vi "Main.vi"() -> ()   [LabVIEW 2018] (continued)
                n1059 = call "DrawROICircle.vi"("old picture"=w1988, "ROI?"=w1976, "Radius (G/S)"=w1975, "Center (G/S)"=w1974, "PicSize"=w1990, "Color"=w1973, "G_max"=w1970, "S_max"=w1968, "G_min"=w1969, "S_min"=w1967) -> ("new picture"=w1987:picture)  [unwired: 9 in]
                n1060 = case shown="\"ROI4\"" w1992 {
                  tunnel: w1993 -> [_ w2002 w2003 w2004 w2005]
                  frame "None" {
                  }
                  frame "ROI1" {
                    "Radius1" <- w2002
                  }
                  frame "ROI2" {
                    "Radius2" <- w2003
                  }
                  frame "ROI3" {
                    "Radius3" <- w2004
                  }
                  frame "ROI4" {
                    "Radius4" <- w2005
                  }
                }
              }
            }
          }
        }
        n1061 = property on="Phasor Plot" class="IntGraph (strict)"(error in=w1891, "PlotImages.Front"=w1892) -> (error out=w1897:errorcluster)  [unwired: 1 in, 1 out]
      }
      event "Phasor Plot": Mouse Up; "ROI1?", "ROI2?", "ROI3?", "ROI4?", "Phasor\nOverlap?", "Refresh Overlap": Value Change {
        n1062 = event-data() -> ()  [unwired: 1 in, 1 out]
        n1063 = local read "ROI Drawing"() -> (w2050:bool)
        n1064 = local read "ROI Select"() -> (w2051:enum16{"None", "ROI1", "ROI2", "ROI3", "ROI4"})
        n1065 = case shown="True" w2050 {
          tunnel: w2051 -> [_ w2076]
          tunnel: w2043 -> [w2073 w2074]
          tunnel: [w2073 w2074] -> w2042
          frame False {
          }
          frame True {
            n1066 = case shown="\"ROI1\"" w2076 {
              frame "None" {
              }
              frame "ROI1" {
                n1067 = local read "Radius1"() -> (w2081:dbl)
                n1068 = Greater Than 0?(x=w2081) -> (x > 0?=w2080:bool)
                n1069 = Select(t=TRUE ("ROI Drawing"), s=w2080, f=FALSE ("ROI Drawing")) -> (s? t:f=w2079:bool)
                n1070 = local write "ROI1?"(w2079) -> ()
              }
              frame "ROI2" {
                n1071 = local read "Radius2"() -> (w2083:dbl)
                n1072 = Greater Than 0?(x=w2083) -> (x > 0?=w2086:bool)
                n1073 = Select(t=TRUE ("ROI Drawing"), s=w2086, f=FALSE ("ROI Drawing")) -> (s? t:f=w2082:bool)
                n1074 = local write "ROI2?"(w2082) -> ()
              }
              frame "ROI3" {
                n1075 = local read "Radius3"() -> (w2089:dbl)
                n1076 = Greater Than 0?(x=w2089) -> (x > 0?=w2090:bool)
                n1077 = Select(t=TRUE ("ROI Drawing"), s=w2090, f=FALSE ("ROI Drawing")) -> (s? t:f=w2088:bool)
                n1078 = local write "ROI3?"(w2088) -> ()
              }
              frame "ROI4" {
                n1079 = local read "Radius4"() -> (w2093:dbl)
                n1080 = Greater Than 0?(x=w2093) -> (x > 0?=w2096:bool)
                n1081 = Select(t=TRUE ("ROI Drawing"), s=w2096, f=FALSE ("ROI Drawing")) -> (s? t:f=w2092:bool)
                n1082 = local write "ROI4?"(w2092) -> ()
              }
            }
            n1083 = local write "ROI Drawing"(FALSE ("ROI Drawing")) -> ()
          }
        }
        n1084 = local read "Radius4"() -> (w2038:dbl)
        n1085 = local read "Center4"() -> (w2035:cluster{dbl, dbl})
        n1086 = local read "Radius2"() -> (w2040:dbl)
        n1087 = local read "Center2"() -> (w2036:cluster{dbl, dbl})
        n1088 = local read "Radius3"() -> (w2039:dbl)
        n1089 = local read "Center3"() -> (w2026:cluster{dbl, dbl})
        n1090 = local read "Radius1"() -> (w2041:dbl)
        n1091 = local read "Center1"() -> (w2037:cluster{dbl, dbl})
        n1092 = local read "PicSize"() -> (w2046:u32)
        n1093 = local read "Color4"() -> (w2031:u32)
        n1094 = local read "Color2"() -> (w2033:u32)
        n1095 = local read "Color3"() -> (w2032:u32)
        n1096 = local read "Color1"() -> (w2034:u32)
        n1097 = local read "ROI4?"() -> (w2016:bool)
        n1098 = local read "ROI3?"() -> (w2017:bool)
        n1099 = local read "ROI1?"() -> (w2019:bool)
        n1100 = local read "ROI2?"() -> (w2018:bool)
        n1101 = Build Array(w2019, w2018, w2017, w2016) -> (w2015:bool[])
        n1102 = Build Array(w2041, w2040, w2039, w2038) -> (w2014:dbl[])
        n1103 = Build Array(w2037, w2036, w2026, w2035) -> (w2013:cluster{dbl, dbl}[])
        n1104 = local read "G_max"() -> (w2025:dbl)
        n1105 = local read "G_min"() -> (w2024:dbl)
        n1106 = local read "S_max"() -> (w2023:dbl)
        n1107 = Build Array(w2034, w2033, w2032, w2031) -> (w2012:u32[])
        n1108 = local read "S_min"() -> (w2022:dbl)
        n1109 = call "Empty Picture"() -> ("empty picture"=w2044:picture)
        n1110 = call "DrawROICircle.vi"("old picture"=w2044, "ROI?"=w2019, "Radius (G/S)"=w2041, "Center (G/S)"=w2037, "PicSize"=w2046, "Color"=w2034, "G_max"=w2025, "S_max"=w2023, "G_min"=w2024, "S_min"=w2022) -> ("new picture"=w2049:picture)  [unwired: 9 in]
        n1111 = call "DrawROICircle.vi"("old picture"=w2049, "ROI?"=w2018, "Radius (G/S)"=w2040, "Center (G/S)"=w2036, "PicSize"=w2046, "Color"=w2033, "G_max"=w2025, "S_max"=w2023, "G_min"=w2024, "S_min"=w2022) -> ("new picture"=w2047:picture)  [unwired: 9 in]
        n1112 = call "DrawROICircle.vi"("old picture"=w2047, "ROI?"=w2017, "Radius (G/S)"=w2039, "Center (G/S)"=w2026, "PicSize"=w2046, "Color"=w2032, "G_max"=w2025, "S_max"=w2023, "G_min"=w2024, "S_min"=w2022) -> ("new picture"=w2048:picture)  [unwired: 9 in]
        n1113 = call "DrawROICircle.vi"("old picture"=w2048, "ROI?"=w2016, "Radius (G/S)"=w2038, "Center (G/S)"=w2035, "PicSize"=w2046, "Color"=w2031, "G_max"=w2025, "S_max"=w2023, "G_min"=w2024, "S_min"=w2022) -> ("new picture"=w2045:picture)  [unwired: 9 in]
        n1114 = local read "Auto Scale?"() -> (w2010:bool)
        n1115 = local read "Max Intensity"() -> (w2009:dbl)
        n1116 = local read "Min Intensity"() -> (w2008:dbl)
        n1117 = control-ref of="Image with Phasors"() -> (w2028:refnum<vi>)
        n1118 = property on="Phasor Plot" class="IntGraph (strict)"(error in=w2042, "PlotImages.Front"=w2045) -> (error out=w2021:errorcluster)  [unwired: 1 in, 1 out]
        n1119 = Bundle(w2015, w2014, w2013, w2012) -> (→"ROI Cluster":T9)  [unwired: 1 in]
        n1120 = local read "V_DC"() -> (w2027:dbl[][])
        n1121 = case shown="True" "Phasor\nOverlap?" {
          tunnel: w2015 -> [_ w2070]
          tunnel: w2014 -> [_ w2069]
          tunnel: w2013 -> [_ w2068]
          tunnel: w2012 -> [_ w2067]
          tunnel: [w2060 w2066] -> w2029
          tunnel: w2028 -> [w2059 w2065]
          tunnel: w2010 -> [w2057 w2064]
          tunnel: w2009 -> [w2056 w2063]
          tunnel: w2008 -> [w2055 w2062]
          tunnel: w2027 -> [w2058 w2061]
          frame False {
            n1122 = call "Array2GrayPic.vi"("Pic Reference"=w2059, "Threshold (min)"=w2055, "Threshold (max)"=w2056, "Auto Scale?"=w2057, "Intensity"=w2058) -> ("Gray Picture"=w2060:picture)  [unwired: 6 in]
          }
          frame True {
            n1123 = local read "G Data"() -> (w2072:dbl[][])
            n1124 = local read "S Data"() -> (w2071:dbl[][])
            n1125 = call "PhasorROI2IMG.vi"("Intensity"=w2061, "Auto Scale?"=w2064, "Threshold (max)"=w2063, "Threshold (min)"=w2062, "G Data"=w2072, "S Data"=w2071, "Pic Reference"=w2065, "ROI? array"=w2070, "Radius array"=w2069, "Center array"=w2068, "Color array"=w2067) -> ("new picture"=w2066:picture)  [unwired: 8 in]
          }
        }
        n1126 = flat-sequence {
          tunnel: [w2054] -> w2020
          tunnel: w2021 -> [w2054]
          frame #0 {
            n1127 = local write "Refresh Overlap"(FALSE ("Fast Scan")) -> ()
          }
        }
        n1128 = local write "Image with Phasors"(w2029) -> ()
      }
      event "Phasor Grids", "G_max", "G_min", "S_max", "S_min", "Phasor Colormap", "Update Phasor": Value Change {
        n1129 = event-data() -> ()  [unwired: 1 in, 1 out]
        n1130 = local read "Phasor Colormap"() -> (w2102:T8)
        n1131 = local read "Max Intensity"() -> (w2100:dbl)
        n1132 = local read "Min Intensity"() -> (w2099:dbl)
        n1133 = local read "Auto Scale?"() -> (w2101:bool)
        n1134 = control-ref of="Phasor Plot"() -> (w2103:refnum<vi>)
        n1135 = local read "Phasor Grids"() -> (w2104:i32)
        n1136 = local read "V_DC"() -> (w2107:dbl[][])
        n1137 = control-ref of="Image with Phasors"() -> (w2116:refnum<vi>)
        n1138 = local read "G Data"() -> (w2106:dbl[][])
        n1139 = local read "S Data"() -> (w2105:dbl[][])
        n1140 = local read "G_max"() -> (w2111:dbl)
        n1141 = local read "S_max"() -> (w2109:dbl)
        n1142 = local read "G_min"() -> (w2110:dbl)
        n1143 = local read "S_min"() -> (w2108:dbl)
        n1144 = call "Array2GrayPic.vi"("Pic Reference"=w2116, "Threshold (min)"=w2099, "Threshold (max)"=w2100, "Auto Scale?"=w2101, "Intensity"=w2107) -> ("Gray Picture"=w2115:picture)  [unwired: 6 in]
        n1145 = call "DrawPhasorPlot.vi"("Intensity"=w2107, "G Data"=w2106, "S Data"=w2105, "Threshold (max)"=w2100, "Threshold (min)"=w2099, "error in"=w2114, "G_max"=w2111, "Auto Scale?"=w2101, "G_min"=w2110, "Phasor Grids"=w2104, "S_max"=w2109, "Reference"=w2103, "S_min"=w2108, "Phasor Colormap"=w2102) -> ("Phasor Plot"=w2112:dbl[][], "error out"=w2113:errorcluster)  [unwired: 4 in]
        n1146 = local write "Image with Phasors"(w2115) -> ()
        n1147 = local write "Phasor Plot"(w2112) -> ()
      }
      event "Load P1": Value Change {
        n1148 = event-data() -> ()  [unwired: 1 in, 1 out]
        n1149 = local read "Measurement Parameters"() -> (w2138:T4)
        n1150 = property on="Composite q1,1" class="Pict"(error in=w2135) -> (error out=w2134:errorcluster, "Draw Area Size"=w2139:T16)  [unwired: 1 in, 1 out]
        n1151 = local read "V_DC"() -> (→"DC,1":dbl[][])
        n1152 = local read "V_IF (pi)"() -> (w2159:dbl[][])
        n1153 = local read "V_IF (0)"() -> (w2158:dbl[][])
        n1154 = local read "V_IF (0.5pi)"() -> (w2157:dbl[][])
        n1155 = local read "V_IF (1.5pi)"() -> (w2156:dbl[][])
        n1156 = Unbundle By Name(w2138) -> ("Pixel Size"=w2137:dbl)
        n1157 = Unbundle By Name(w2139) -> ("Width"=w2140:u32)
        n1158 = To Single Precision Float(number=w2140) -> (single precision float=w2142:sgl)
        n1159 = To Single Precision Float(number=w2137) -> (single precision float=w2141:sgl)
        n1160 = Divide(x=w2142, y=w2141) -> (x/y=w2136:sgl)
        n1161 = Subtract(x=w2159, y=w2158) -> (x-y=w2151:dbl[][])
        n1162 = Subtract(x=w2157, y=w2156) -> (x-y=w2152:dbl[][])
        n1163 = property on="Composite q1,1" class="Pict"(error in=w2134, "ZoomFactor"=w2136) -> (error out=w2130:errorcluster)  [unwired: 1 in, 1 out]
        n1164 = local read "tau_max (s)"() -> (w2132:dbl)
        n1165 = local read "tau_min (s)"() -> (w2131:dbl)
        n1166 = Square(x=w2151) -> (x^2=w2155:dbl[][])
        n1167 = Square(x=w2152) -> (x^2=w2154:dbl[][])
        n1168 = Divide(x=w2151, y=w2152) -> (x/y=w2150:dbl[][])
        n1169 = local read "LaserRepRate (Hz)"() -> (w2118:dbl)
        n1170 = Add(x=w2155, y=w2154) -> (x+y=w2153:dbl[][])
        n1171 = Inverse Tangent(1:w2150) -> (0:w2148:dbl[][])
        "Angle q1,1" <- w2148
        n1172 = property on="Lifetime q1,1" class="IntGraph (strict)"(error in=w2130, "ZScale.Minimum"=w2131) -> (error out=w2129:errorcluster)  [unwired: 1 in, 1 out]
        n1173 = Square Root(x=w2153) -> (sqrt(x)=w2127:dbl[][])
        "Mag q1,1" <- w2127
        n1174 = Tangent(1:w2148) -> (0:w2147:dbl[][])
        n1175 = Multiply(x=w2118, y=6.283185307179586) -> (x*y=w2146:dbl)
        n1176 = local read "Custom Mag?"() -> (w2128:bool)
        n1177 = Divide(x=w2147, y=w2146) -> (x/y=w2145:dbl[][])
        n1178 = property on="Lifetime q1,1" class="IntGraph (strict)"(error in=w2129, "ZScale.Maximum"=w2132) -> (error out=w2126:errorcluster)  [unwired: 1 in, 1 out]
        n1179 = Negate(x=w2145) -> (-x=w2143:dbl[][])
        "Lifetime q1,1" <- w2143
        n1180 = case shown="True" w2128 {
          tunnel: w2127 -> [w2163 _]
          tunnel: [w2162 "q1,1max"] -> w2122
          tunnel: [w2161 "q1,1min"] -> w2123
          frame False {
            n1181 = Array Max & Min(array=w2163) -> (max value=w2162:dbl, min value=w2161:dbl)  [unwired: 2 out]
          }
          frame True {
          }
        }
        n1182 = call "HSVCombIntensityLifetime.vi"("min_intensity"=w2123, "Auto Scale?"=TRUE ("External Bound Intensity Value?"), "max_intensity"=w2122, "lifetime_max (s)"=w2132, "lifetime_min (s)"=w2131, "Lifetime image"=w2143, "Intensity image"=w2127) -> ("HSV to RGB Picture"=→"Composite q1,1":picture)  [unwired: 1 in, 3 out]
        n1183 = property on="Mag q1,1" class="IntGraph (strict)"(error in=w2126, "ZScale.Minimum"=w2123) -> (error out=w2125:errorcluster)  [unwired: 1 in, 1 out]
        n1184 = property on="Mag q1,1" class="IntGraph (strict)"(error in=w2125, "ZScale.Maximum"=w2122) -> (error out=w2124:errorcluster)  [unwired: 1 in, 1 out]
      }
      event "Load P2": Value Change {
        n1185 = event-data() -> ()  [unwired: 1 in, 1 out]
        n1186 = local read "Measurement Parameters"() -> (w2186:T4)
        n1187 = property on="Composite q1,2" class="Pict"(error in=w2185) -> (error out=w2184:errorcluster, "Draw Area Size"=w2183:T16)  [unwired: 1 in, 1 out]
        n1188 = Unbundle By Name(w2186) -> ("Pixel Size"=w2187:dbl)
        n1189 = local read "V_IF (pi)"() -> (w2201:dbl[][])
        n1190 = local read "V_IF (0)"() -> (w2200:dbl[][])
        n1191 = local read "V_IF (0.5pi)"() -> (w2199:dbl[][])
        n1192 = local read "V_IF (1.5pi)"() -> (w2198:dbl[][])
        n1193 = local read "V_DC"() -> (→"DC,2":dbl[][])
        n1194 = Unbundle By Name(w2183) -> ("Width"=w2188:u32)
        n1195 = To Single Precision Float(number=w2188) -> (single precision float=w2190:sgl)
        n1196 = To Single Precision Float(number=w2187) -> (single precision float=w2189:sgl)
        n1197 = Divide(x=w2190, y=w2189) -> (x/y=w2182:sgl)
        n1198 = Subtract(x=w2201, y=w2200) -> (x-y=w2203:dbl[][])
        n1199 = Subtract(x=w2199, y=w2198) -> (x-y=w2204:dbl[][])
        n1200 = property on="Composite q1,2" class="Pict"(error in=w2184, "ZoomFactor"=w2182) -> (error out=w2177:errorcluster)  [unwired: 1 in, 1 out]
        n1201 = local read "tau_max (s)"() -> (w2180:dbl)
        n1202 = local read "tau_min (s)"() -> (w2181:dbl)
        n1203 = Square(x=w2203) -> (x^2=w2207:dbl[][])
        n1204 = Square(x=w2204) -> (x^2=w2206:dbl[][])
        n1205 = Divide(x=w2203, y=w2204) -> (x/y=w2202:dbl[][])
        n1206 = property on="Lifetime q1,2" class="IntGraph (strict)"(error in=w2177, "ZScale.Minimum"=w2181) -> (error out=w2176:errorcluster)  [unwired: 1 in, 1 out]
        n1207 = local read "LaserRepRate (Hz)"() -> (w2166:dbl)
        n1208 = Add(x=w2207, y=w2206) -> (x+y=w2205:dbl[][])
        n1209 = Inverse Tangent(1:w2202) -> (0:w2170:dbl[][])
        "Angle q1,2" <- w2170
        n1210 = local read "Custom Mag?"() -> (w2179:bool)
        n1211 = property on="Lifetime q1,2" class="IntGraph (strict)"(error in=w2176, "ZScale.Maximum"=w2180) -> (error out=w2175:errorcluster)  [unwired: 1 in, 1 out]
        n1212 = Square Root(x=w2205) -> (sqrt(x)=w2178:dbl[][])
        "Mag q1,2" <- w2178
        n1213 = Tangent(1:w2170) -> (0:w2196:dbl[][])
        n1214 = Multiply(x=w2166, y=6.283185307179586) -> (x*y=w2195:dbl)
        n1215 = case shown="True" w2179 {
          tunnel: w2178 -> [w2211 _]
          tunnel: [w2210 "q1,2max"] -> w2172
          tunnel: [w2209 "q1,2min"] -> w2171
          frame False {
            n1216 = Array Max & Min(array=w2211) -> (max value=w2210:dbl, min value=w2209:dbl)  [unwired: 2 out]
          }
          frame True {
          }
        }
        n1217 = Divide(x=w2196, y=w2195) -> (x/y=w2194:dbl[][])
        n1218 = Negate(x=w2194) -> (-x=w2192:dbl[][])
        "Lifetime q1,2" <- w2192
        n1219 = call "HSVCombIntensityLifetime.vi"("min_intensity"=w2171, "Auto Scale?"=TRUE ("External Bound Intensity Value?"), "max_intensity"=w2172, "lifetime_max (s)"=w2180, "lifetime_min (s)"=w2181, "Lifetime image"=w2192, "Intensity image"=w2178) -> ("HSV to RGB Picture"=→"Composite q1,2":picture)  [unwired: 1 in, 3 out]
        n1220 = property on="Mag q1,2" class="IntGraph (strict)"(error in=w2175, "ZScale.Minimum"=w2171) -> (error out=w2174:errorcluster)  [unwired: 1 in, 1 out]
        n1221 = property on="Mag q1,2" class="IntGraph (strict)"(error in=w2174, "ZScale.Maximum"=w2172) -> (error out=w2173:errorcluster)  [unwired: 1 in, 1 out]
      }
      event "Two-Step GSOS": Value Change {
        n1222 = event-data() -> ()  [unwired: 1 in, 1 out]
        n1223 = local read "Measurement Parameters"() -> (w2237:T4)
        n1224 = property on="Composite GSOS" class="Pict"(error in=w2239) -> (error out=w2238:errorcluster, "Draw Area Size"=w2241:T16)  [unwired: 1 in, 1 out]
        n1225 = local read "Mag q1,1"() -> (w2262:dbl[][])
        n1226 = local read "Angle q1,2"() -> (w2224:dbl[][])
        n1227 = local read "Angle q1,1"() -> (w2225:dbl[][])
        n1228 = local read "Mag q1,2"() -> (w2261:dbl[][])
        n1229 = local read "DC,1"() -> (w2220:dbl[][])
        n1230 = local read "DC,2"() -> (w2222:dbl[][])
        n1231 = Unbundle By Name(w2237) -> ("Pixel Size"=w2242:dbl)
        n1232 = Unbundle By Name(w2241) -> ("Width"=w2243:u32)
        n1233 = To Single Precision Float(number=w2243) -> (single precision float=w2245:sgl)
        n1234 = To Single Precision Float(number=w2242) -> (single precision float=w2244:sgl)
        n1235 = Divide(x="P1 Power (au)", y="P2 Power (au)") -> (x/y=w2258:dbl)
        n1236 = Polar To Complex(1:w2224, 2:w2261) -> (0:w2255:cdb[][])
        n1237 = Polar To Complex(1:w2225, 2:w2262) -> (0:w2256:cdb[][])
        n1238 = Square(x=w2258) -> (x^2=w2257:dbl)
        n1239 = Divide(x=w2245, y=w2244) -> (x/y=w2240:sgl)
        n1240 = Negate(x=w2257) -> (-x=w2219:dbl)
        n1241 = property on="Composite GSOS" class="Pict"(error in=w2238, "ZoomFactor"=w2240) -> (error out=w2234:errorcluster)  [unwired: 1 in, 1 out]
        n1242 = To Double Precision Complex(1:w2219) -> (0:w2221:cdb)
        n1243 = local read "tau_max (s)"() -> (w2235:dbl)
        n1244 = local read "tau_min (s)"() -> (w2236:dbl)
        n1245 = Multiply(x=w2255, y=w2221) -> (x*y=w2254:cdb[][])
        n1246 = Multiply(x=w2222, y=w2219) -> (x*y=w2218:dbl[][])
        n1247 = Add(x=w2220, y=w2218) -> (x+y=→"DC,SOS":dbl[][])
        n1248 = Add(x=w2256, y=w2254) -> (x+y=w2253:cdb[][])
        n1249 = property on="Lifetime GSOS" class="IntGraph (strict)"(error in=w2234, "ZScale.Minimum"=w2236) -> (error out=w2233:errorcluster)  [unwired: 1 in, 1 out]
        n1250 = local read "LaserRepRate (Hz)"() -> (w2214:dbl)
        n1251 = Complex To Polar(r * e^(i*theta)=w2253) -> (r=w2231:dbl[][], theta=w2223:dbl[][])
        "Mag GSOS" <- w2231
        "Angle GSOS" <- w2223
        n1252 = local read "Custom Mag?"() -> (w2232:bool)
        n1253 = property on="Lifetime GSOS" class="IntGraph (strict)"(error in=w2233, "ZScale.Maximum"=w2235) -> (error out=w2230:errorcluster)  [unwired: 1 in, 1 out]
        n1254 = Tangent(1:w2223) -> (0:w2251:dbl[][])
        n1255 = case shown="True" w2232 {
          tunnel: w2231 -> [w2266 _]
          tunnel: [w2265 "qGSmax"] -> w2227
          tunnel: [w2264 "qGSmin"] -> w2226
          frame False {
            n1256 = Array Max & Min(array=w2266) -> (max value=w2265:dbl, min value=w2264:dbl)  [unwired: 2 out]
          }
          frame True {
          }
        }
        n1257 = Multiply(x=w2214, y=6.283185307179586) -> (x*y=w2250:dbl)
        n1258 = Divide(x=w2251, y=w2250) -> (x/y=w2249:dbl[][])
        n1259 = Negate(x=w2249) -> (-x=w2247:dbl[][])
        "Lifetime GSOS" <- w2247
        n1260 = call "HSVCombIntensityLifetime.vi"("min_intensity"=w2226, "Auto Scale?"=TRUE ("External Bound Intensity Value?"), "max_intensity"=w2227, "lifetime_max (s)"=w2235, "lifetime_min (s)"=w2236, "Lifetime image"=w2247, "Intensity image"=w2231) -> ("HSV to RGB Picture"=→"Composite GSOS":picture)  [unwired: 1 in, 3 out]
        n1261 = property on="Mag GSOS" class="IntGraph (strict)"(error in=w2230, "ZScale.Minimum"=w2226) -> (error out=w2229:errorcluster)  [unwired: 1 in, 1 out]
        n1262 = property on="Mag GSOS" class="IntGraph (strict)"(error in=w2229, "ZScale.Maximum"=w2227) -> (error out=w2228:errorcluster)  [unwired: 1 in, 1 out]
      }
      event "Export GSOS Images": Value Change {
        n1263 = event-data() -> ()  [unwired: 1 in, 1 out]
        n1264 = local read "Current Directory (2D)?"() -> (w2349:bool)
        n1265 = local read "Mag q1,1"() -> (w2315:dbl[][])
        n1266 = local read "Mag q1,2"() -> (w2314:dbl[][])
        n1267 = local read "Mag GSOS"() -> (w2313:dbl[][])
        n1268 = case shown="True" w2349 {
          tunnel: [w2373 w2374] -> w2348
          frame False {
            n1269 = local read "Save Directory (2D)"() -> (w2373:path)
          }
          frame True {
            n1270 = Current VI's Path() -> (path=w2375:path)
            n1271 = Strip Path(path=w2375) -> (stripped path=w2374:path)  [unwired: 1 out]
          }
        }
        n1272 = local read "Experiment Name (2D)"() -> (w2347:string)
        n1273 = local read "File Name (2D)"() -> (w2322:string)
        n1274 = case shown="True" "Custom Mag?" {
          tunnel: w2315 -> [w2366 _]
          tunnel: [w2365 w2372] -> w2312
          tunnel: [w2364 w2371] -> w2311
          tunnel: [w2362 w2370] -> w2310
          tunnel: [w2363 w2369] -> w2309
          tunnel: [w2361 w2368] -> w2308
          tunnel: [w2360 w2367] -> w2307
          tunnel: w2314 -> [w2359 _]
          tunnel: w2313 -> [w2358 _]
          frame False {
            n1275 = Array Max & Min(array=w2366) -> (max value=w2365:dbl, min value=w2364:dbl)  [unwired: 2 out]
            n1276 = Array Max & Min(array=w2359) -> (max value=w2362:dbl, min value=w2363:dbl)  [unwired: 2 out]
            n1277 = Array Max & Min(array=w2358) -> (max value=w2361:dbl, min value=w2360:dbl)  [unwired: 2 out]
          }
          frame True {
            n1278 = local read "q1,1max"() -> (w2372:dbl)
            n1279 = local read "q1,1min"() -> (w2371:dbl)
            n1280 = local read "q1,2max"() -> (w2370:dbl)
            n1281 = local read "q1,2min"() -> (w2369:dbl)
            n1282 = local read "qGSmax"() -> (w2368:dbl)
            n1283 = local read "qGSmin"() -> (w2367:dbl)
          }
        }
        n1284 = Concatenate Strings(w2347, "_" ("string"), "GSOS" ("string")) -> (w2354:string)
        n1285 = Build Path(base path=w2348, name or relative path=w2354) -> (appended path=w2357:path)
        n1286 = call <vilib>:"Check if File or Folder Exists.vi"("error in (no error)"=w2351, "path"=w2357) -> ("error out"=w2356:errorcluster, "file or folder exists?"=w2346:bool, "dup path"=w2355:path)  [unwired: 7 in]
        n1287 = local read "Lifetime q1,1"() -> (w2332:dbl[][])
        n1288 = case shown="False" w2346 {
          tunnel: w2356 -> [w2379 w2380]
          tunnel: [w2378 w2380] -> w2300
          tunnel: [w2377 w2381] -> w2321
          tunnel: w2355 -> [w2376 w2381]
          frame False {
            n1289 = Create Folder(path (use dialog)=w2376, error in=w2379) -> (created path=w2377:path, error out=w2378:errorcluster)  [unwired: 1 in, 1 out]
          }
          frame True {
          }
        }
        n1290 = local read "Angle q1,1"() -> (w2306:dbl[][])
        n1291 = local read "DC,1"() -> (w2303:dbl[][])
        n1292 = call "HSVCombIntensityLifetime.vi"("min_intensity"=w2311, "Auto Scale?"=FALSE ("External Bound Intensity Value?"), "max_intensity"=w2312, "lifetime_max (s)"="tau_max (s)", "lifetime_min (s)"="tau_min (s)", "Lifetime image"=w2332, "Intensity image"=w2315) -> ("HSV to RGB Picture"=w2334:picture)  [unwired: 1 in, 3 out]
        n1293 = call "Save2RealTIF.vi"("min_value"=w2311, "Specify Range?"=TRUE ("Bound Pixel Value?"), "max_value"=w2312, "Time Stamp?"=FALSE, "File Name Prefix"=w2322, "error in"=w2300, "Identify Name"="q1_Mag" ("string"), "Data 2D Array"=w2315, "Parent Directory"=w2321) -> ("error out"=w2299:errorcluster)  [unwired: 1 in, 1 out]
        n1294 = local read "Angle q1,2"() -> (w2305:dbl[][])
        n1295 = local read "DC,2"() -> (w2302:dbl[][])
        n1296 = local read "Lifetime q1,2"() -> (w2327:dbl[][])
        n1297 = call "HSVCombIntensityLifetime.vi"("min_intensity"=w2309, "Auto Scale?"=FALSE ("External Bound Intensity Value?"), "max_intensity"=w2310, "lifetime_max (s)"="tau_max (s)", "lifetime_min (s)"="tau_min (s)", "Lifetime image"=w2327, "Intensity image"=w2314) -> ("HSV to RGB Picture"=w2330:picture)  [unwired: 1 in, 3 out]
        n1298 = call "Save2RealTIF.vi"("min_value"=w2309, "Specify Range?"=TRUE ("Bound Pixel Value?"), "max_value"=w2310, "Time Stamp?"=FALSE, "File Name Prefix"=w2322, "error in"=w2299, "Identify Name"="q2_Mag" ("string"), "Data 2D Array"=w2314, "Parent Directory"=w2321) -> ("error out"=w2298:errorcluster)  [unwired: 1 in, 1 out]
        n1299 = local read "Angle GSOS"() -> (w2304:dbl[][])
        n1300 = local read "DC,SOS"() -> (w2301:dbl[][])
        n1301 = local read "Lifetime GSOS"() -> (w2320:dbl[][])
        n1302 = call "HSVCombIntensityLifetime.vi"("min_intensity"=w2307, "Auto Scale?"=FALSE ("External Bound Intensity Value?"), "max_intensity"=w2308, "lifetime_max (s)"="tau_max (s)", "lifetime_min (s)"="tau_min (s)", "Lifetime image"=w2320, "Intensity image"=w2313) -> ("HSV to RGB Picture"=w2325:picture)  [unwired: 1 in, 3 out]
        n1303 = call "Save2RealTIF.vi"("min_value"=w2307, "Specify Range?"=TRUE ("Bound Pixel Value?"), "max_value"=w2308, "Time Stamp?"=FALSE, "File Name Prefix"=w2322, "error in"=w2298, "Identify Name"="q2GSOS_Mag" ("string"), "Data 2D Array"=w2313, "Parent Directory"=w2321) -> ("error out"=w2297:errorcluster)  [unwired: 1 in, 1 out]
        n1304 = call "Save2RealTIF.vi"("Specify Range?"=FALSE ("Bound Pixel Value?"), "Time Stamp?"=FALSE, "File Name Prefix"=w2322, "error in"=w2297, "Identify Name"="q1_Angle" ("string"), "Data 2D Array"=w2306, "Parent Directory"=w2321) -> ("error out"=w2296:errorcluster)  [unwired: 3 in, 1 out]
        n1305 = call "Save2RealTIF.vi"("Specify Range?"=FALSE ("Bound Pixel Value?"), "Time Stamp?"=FALSE, "File Name Prefix"=w2322, "error in"=w2296, "Identify Name"="q2_Angle" ("string"), "Data 2D Array"=w2305, "Parent Directory"=w2321) -> ("error out"=w2295:errorcluster)  [unwired: 3 in, 1 out]
        n1306 = call "Save2RealTIF.vi"("Specify Range?"=FALSE ("Bound Pixel Value?"), "Time Stamp?"=FALSE, "File Name Prefix"=w2322, "error in"=w2295, "Identify Name"="q2GSOS_Angle" ("string"), "Data 2D Array"=w2304, "Parent Directory"=w2321) -> ("error out"=w2294:errorcluster)  [unwired: 3 in, 1 out]
        n1307 = call "Save2RealTIF.vi"("Specify Range?"=FALSE ("Bound Pixel Value?"), "Time Stamp?"=FALSE, "File Name Prefix"=w2322, "error in"=w2294, "Identify Name"="DC_1" ("string"), "Data 2D Array"=w2303, "Parent Directory"=w2321) -> ("error out"=w2293:errorcluster)  [unwired: 3 in, 1 out]
        n1308 = call "Save2RealTIF.vi"("Specify Range?"=FALSE ("Bound Pixel Value?"), "Time Stamp?"=FALSE, "File Name Prefix"=w2322, "error in"=w2293, "Identify Name"="DC_2" ("string"), "Data 2D Array"=w2302, "Parent Directory"=w2321) -> ("error out"=w2292:errorcluster)  [unwired: 3 in, 1 out]
        n1309 = call "Save2RealTIF.vi"("Specify Range?"=FALSE ("Bound Pixel Value?"), "Time Stamp?"=FALSE, "File Name Prefix"=w2322, "error in"=w2292, "Identify Name"="DC_SOS" ("string"), "Data 2D Array"=w2301, "Parent Directory"=w2321) -> ("error out"=w2336:errorcluster)  [unwired: 3 in, 1 out]
        n1310 = call "Save2ColorPNG.vi"("Time Stamp?"=FALSE, "File Name Prefix"=w2322, "error in"=w2336, "Identify Name"="q1_Composite" ("string"), "Data Picture"=w2334, "Parent Directory"=w2321) -> ("error out"=w2328:errorcluster)  [unwired: 4 in, 1 out]
        n1311 = call "Save2ColorPNG.vi"("Time Stamp?"=FALSE, "File Name Prefix"=w2322, "error in"=w2328, "Identify Name"="q2_Composite" ("string"), "Data Picture"=w2330, "Parent Directory"=w2321) -> ("error out"=w2323:errorcluster)  [unwired: 4 in, 1 out]
        n1312 = call "Save2ColorPNG.vi"("Time Stamp?"=FALSE, "File Name Prefix"=w2322, "error in"=w2323, "Identify Name"="q2GSOS_Composite" ("string"), "Data Picture"=w2325, "Parent Directory"=w2321) -> ("error out"=w2319:errorcluster)  [unwired: 4 in, 1 out]
      }
      event "tau_max (s)", "tau_min (s)", "q1,1max", "q1,1min", "q1,2max", "q1,2min", "qGSmax", "qGSmin", "Custom Mag?": Value Change {
        n1313 = event-data() -> ()  [unwired: 1 in, 1 out]
        n1314 = local read "tau_max (s)"() -> (w2386:dbl)
        n1315 = local read "tau_min (s)"() -> (w2387:dbl)
        n1316 = property on="Lifetime q1,1" class="IntGraph (strict)"(error in=w2417, "ZScale.Minimum"=w2387) -> (error out=w2416:errorcluster)  [unwired: 1 in, 1 out]
        n1317 = property on="Lifetime q1,1" class="IntGraph (strict)"(error in=w2416, "ZScale.Maximum"=w2386) -> (error out=w2415:errorcluster)  [unwired: 1 in, 1 out]
        n1318 = local read "Lifetime GSOS"() -> (w2385:dbl[][])
        n1319 = local read "Custom Mag?"() -> (w2418:bool)
        n1320 = local read "Lifetime q1,2"() -> (w2394:dbl[][])
        n1321 = local read "Lifetime q1,1"() -> (w2393:dbl[][])
        n1322 = local read "Mag GSOS"() -> (w2388:dbl[][])
        n1323 = local read "Mag q1,2"() -> (w2395:dbl[][])
        n1324 = local read "Mag q1,1"() -> (w2402:dbl[][])
        n1325 = property on="Lifetime q1,2" class="IntGraph (strict)"(error in=w2415, "ZScale.Minimum"=w2387) -> (error out=w2414:errorcluster)  [unwired: 1 in, 1 out]
        n1326 = case shown="True" w2418 {
          tunnel: w2402 -> [w2427 _]
          tunnel: [w2426 w2433] -> w2401
          tunnel: [w2425 w2432] -> w2400
          tunnel: [w2423 w2431] -> w2397
          tunnel: [w2424 w2430] -> w2396
          tunnel: [w2422 w2429] -> w2390
          tunnel: [w2421 w2428] -> w2389
          tunnel: w2395 -> [w2420 _]
          tunnel: w2388 -> [w2419 _]
          frame False {
            n1327 = Array Max & Min(array=w2427) -> (max value=w2426:dbl, min value=w2425:dbl)  [unwired: 2 out]
            n1328 = Array Max & Min(array=w2420) -> (max value=w2423:dbl, min value=w2424:dbl)  [unwired: 2 out]
            n1329 = Array Max & Min(array=w2419) -> (max value=w2422:dbl, min value=w2421:dbl)  [unwired: 2 out]
          }
          frame True {
            n1330 = local read "q1,1max"() -> (w2433:dbl)
            n1331 = local read "q1,1min"() -> (w2432:dbl)
            n1332 = local read "q1,2max"() -> (w2431:dbl)
            n1333 = local read "q1,2min"() -> (w2430:dbl)
            n1334 = local read "qGSmax"() -> (w2429:dbl)
            n1335 = local read "qGSmin"() -> (w2428:dbl)
          }
        }
        n1336 = property on="Lifetime q1,2" class="IntGraph (strict)"(error in=w2414, "ZScale.Maximum"=w2386) -> (error out=w2413:errorcluster)  [unwired: 1 in, 1 out]
        n1337 = property on="Lifetime GSOS" class="IntGraph (strict)"(error in=w2413, "ZScale.Minimum"=w2387) -> (error out=w2412:errorcluster)  [unwired: 1 in, 1 out]
        n1338 = call "HSVCombIntensityLifetime.vi"("min_intensity"=w2400, "Auto Scale?"=TRUE ("External Bound Intensity Value?"), "max_intensity"=w2401, "lifetime_max (s)"=w2386, "lifetime_min (s)"=w2387, "Lifetime image"=w2393, "Intensity image"=w2402) -> ("HSV to RGB Picture"=w2399:picture)  [unwired: 1 in, 3 out]
        n1339 = property on="Lifetime GSOS" class="IntGraph (strict)"(error in=w2412, "ZScale.Maximum"=w2386) -> (error out=w2411:errorcluster)  [unwired: 1 in, 1 out]
        n1340 = call "HSVCombIntensityLifetime.vi"("min_intensity"=w2396, "Auto Scale?"=TRUE ("External Bound Intensity Value?"), "max_intensity"=w2397, "lifetime_max (s)"=w2386, "lifetime_min (s)"=w2387, "Lifetime image"=w2394, "Intensity image"=w2395) -> ("HSV to RGB Picture"=w2392:picture)  [unwired: 1 in, 3 out]
        n1341 = call "HSVCombIntensityLifetime.vi"("min_intensity"=w2389, "Auto Scale?"=TRUE ("External Bound Intensity Value?"), "max_intensity"=w2390, "lifetime_max (s)"=w2386, "lifetime_min (s)"=w2387, "Lifetime image"=w2385, "Intensity image"=w2388) -> ("HSV to RGB Picture"=w2384:picture)  [unwired: 1 in, 3 out]
        n1342 = property on="Mag q1,1" class="IntGraph (strict)"(error in=w2411, "ZScale.Minimum"=w2400) -> (error out=w2410:errorcluster)  [unwired: 1 in, 1 out]
        n1343 = local write "Composite GSOS"(w2384) -> ()
        n1344 = local write "Composite q1,1"(w2399) -> ()
        n1345 = local write "Composite q1,2"(w2392) -> ()
        n1346 = property on="Mag q1,1" class="IntGraph (strict)"(error in=w2410, "ZScale.Maximum"=w2401) -> (error out=w2409:errorcluster)  [unwired: 1 in, 1 out]
        n1347 = property on="Mag q1,2" class="IntGraph (strict)"(error in=w2409, "ZScale.Minimum"=w2396) -> (error out=w2408:errorcluster)  [unwired: 1 in, 1 out]
        n1348 = property on="Mag q1,2" class="IntGraph (strict)"(error in=w2408, "ZScale.Maximum"=w2397) -> (error out=w2407:errorcluster)  [unwired: 1 in, 1 out]
        n1349 = property on="Mag GSOS" class="IntGraph (strict)"(error in=w2407, "ZScale.Minimum"=w2389) -> (error out=w2406:errorcluster)  [unwired: 1 in, 1 out]
        n1350 = property on="Mag GSOS" class="IntGraph (strict)"(error in=w2406, "ZScale.Maximum"=w2390) -> (error out=w2405:errorcluster)  [unwired: 1 in, 1 out]
      }
      event "Save 2D Images": Value Change {
        n1351 = event-data() -> ()  [unwired: 1 in, 1 out]
        n1352 = local read "Current Directory (2D)?"() -> (w2485:bool)
        n1353 = local read "V_DC"() -> (w2441:dbl[][])
        n1354 = local read "Auto Scale?"() -> (w2440:bool)
        n1355 = local read "Current 2D Time-Lapse Meas"() -> (w2443:i32)
        n1356 = case shown="False" w2485 {
          tunnel: ["Save Directory (2D)" w2522] -> w2450
          frame False {
          }
          frame True {
            n1357 = Current VI's Path() -> (path=w2523:path)
            n1358 = Strip Path(path=w2523) -> (stripped path=w2522:path)  [unwired: 1 out]
          }
        }
        n1359 = local read "DC&1w Lifetime (s)"() -> (w2487:dbl[][])
        n1360 = local read "Max Lifetime (s)"() -> (w2488:dbl)
        n1361 = local read "Min Lifetime (s)"() -> (w2489:dbl)
        n1362 = local read "1w Lifetime (s)"() -> (w2486:dbl[][])
        n1363 = local read "V_IF (0.5pi)"() -> (w2469:dbl[][])
        n1364 = local read "V_IF (1.5pi)"() -> (w2467:dbl[][])
        n1365 = local read "V_IF (pi)"() -> (w2468:dbl[][])
        n1366 = local read "V_IF (0)"() -> (w2480:dbl[][])
        n1367 = local read "G Data"() -> (w2448:dbl[][])
        n1368 = local read "S Data"() -> (w2447:dbl[][])
        n1369 = case shown="False" w2440 {
          tunnel: [w2515 w2517] -> w2439
          tunnel: [w2514 w2516] -> w2438
          tunnel: w2441 -> [_ w2518]
          frame False {
            n1370 = local read "Max Intensity"() -> (w2515:dbl)
            n1371 = local read "Min Intensity"() -> (w2514:dbl)
          }
          frame True {
            n1372 = Array Max & Min(array=w2518) -> (max value=w2517:dbl, min value=w2516:dbl)  [unwired: 2 out]
          }
        }
        n1373 = Number To Decimal String(number=w2443) -> (decimal integer string=w2436:string)  [unwired: 1 in]
        n1374 = call "SaveMatrix.vi"("Experiment Name"="Experiment Name (2D)", "Identify Name"="I" ("string"), "Data"=w2441, "matrix_max"=w2439, "matrix_min"=w2438, "error in"=w2466, "File Name"="File Name (2D)", "Index Name"=w2436, "path"=w2450, "Specify Range?"=FALSE ("Bound Pixel Value?"), "Enable?"="Intensity?", "Crop Pixels"="Crop Pixels", "Time Stamp?"="Time Stamp?") -> ("error out"=w2498:errorcluster)  [unwired: 5 in, 1 out]
        n1375 = call "SaveMatrix.vi"("Experiment Name"="Experiment Name (2D)", "Identify Name"="Tau1" ("string"), "Data"=w2486, "error in"=w2498, "File Name"="File Name (2D)", "Index Name"=w2436, "path"=w2450, "Specify Range?"=FALSE ("Bound Pixel Value?"), "Enable?"="1w Lifetime?", "Crop Pixels"="Crop Pixels", "Time Stamp?"="Time Stamp?") -> ("error out"=w2499:errorcluster)  [unwired: 7 in, 1 out]
        n1376 = call "SaveMatrix.vi"("Experiment Name"="Experiment Name (2D)", "Identify Name"="Tau01" ("string"), "Data"=w2487, "error in"=w2499, "File Name"="File Name (2D)", "Index Name"=w2436, "path"=w2450, "Specify Range?"=FALSE ("Bound Pixel Value?"), "Enable?"="DC&1w Lifetime?", "Crop Pixels"="Crop Pixels", "Time Stamp?"="Time Stamp?") -> ("error out"=w2501:errorcluster)  [unwired: 7 in, 1 out]
        n1377 = call "SaveHSVComb.vi"("File Name"="File Name (2D)", "Intensity"=w2441, "intensity_max"=w2439, "intensity_min"=w2438, "Lifetime"=w2486, "lifetime_max (s)"=w2488, "lifetime_min (s)"=w2489, "error in"=w2501, "Experiment Name"="Experiment Name (2D)", "Index Name"=w2436, "Identify Name"="Comp1" ("string"), "Enable?"="1w Composite?", "path"=w2450, "Crop Pixels"="Crop Pixels", "Time Stamp?"="Time Stamp?") -> ("error out"=w2503:errorcluster)  [unwired: 11 in, 1 out]
        n1378 = call "SaveHSVComb.vi"("File Name"="File Name (2D)", "Intensity"=w2441, "intensity_max"=w2439, "intensity_min"=w2438, "Lifetime"=w2487, "lifetime_max (s)"=w2488, "lifetime_min (s)"=w2489, "error in"=w2503, "Experiment Name"="Experiment Name (2D)", "Index Name"=w2436, "Identify Name"="Comp01" ("string"), "Enable?"="DC&1w Composite?", "path"=w2450, "Crop Pixels"="Crop Pixels", "Time Stamp?"="Time Stamp?") -> ("error out"=w2505:errorcluster)  [unwired: 11 in, 1 out]
        n1379 = call "SaveMatrix.vi"("Experiment Name"="Experiment Name (2D)", "Identify Name"="G" ("string"), "Data"=w2448, "error in"=w2505, "File Name"="File Name (2D)", "Index Name"=w2436, "path"=w2450, "Specify Range?"=FALSE ("Bound Pixel Value?"), "Enable?"="G?", "Crop Pixels"="Crop Pixels", "Time Stamp?"="Time Stamp?") -> ("error out"=w2506:errorcluster)  [unwired: 7 in, 1 out]
        n1380 = call "SaveMatrix.vi"("Experiment Name"="Experiment Name (2D)", "Identify Name"="S" ("string"), "Data"=w2447, "error in"=w2506, "File Name"="File Name (2D)", "Index Name"=w2436, "path"=w2450, "Specify Range?"=FALSE ("Bound Pixel Value?"), "Enable?"="S?", "Crop Pixels"="Crop Pixels", "Time Stamp?"="Time Stamp?") -> ("error out"=w2481:errorcluster)  [unwired: 7 in, 1 out]
        n1381 = call "SaveMatrix.vi"("Experiment Name"="Experiment Name (2D)", "Identify Name"="Mix1" ("string"), "Data"=w2480, "error in"=w2481, "File Name"="File Name (2D)", "Index Name"=w2436, "path"=w2450, "Specify Range?"=FALSE ("Bound Pixel Value?"), "Enable?"="4 Mix?", "Crop Pixels"="Crop Pixels", "Time Stamp?"="Time Stamp?") -> ("error out"=w2473:errorcluster)  [unwired: 7 in, 1 out]
        n1382 = call "SaveMatrix.vi"("Experiment Name"="Experiment Name (2D)", "Identify Name"="Mix2" ("string"), "Data"=w2469, "error in"=w2473, "File Name"="File Name (2D)", "Index Name"=w2436, "path"=w2450, "Specify Range?"=FALSE ("Bound Pixel Value?"), "Enable?"="4 Mix?", "Crop Pixels"="Crop Pixels", "Time Stamp?"="Time Stamp?") -> ("error out"=w2472:errorcluster)  [unwired: 7 in, 1 out]
        n1383 = call "SaveMatrix.vi"("Experiment Name"="Experiment Name (2D)", "Identify Name"="Mix3" ("string"), "Data"=w2468, "error in"=w2472, "File Name"="File Name (2D)", "Index Name"=w2436, "path"=w2450, "Specify Range?"=FALSE ("Bound Pixel Value?"), "Enable?"="4 Mix?", "Crop Pixels"="Crop Pixels", "Time Stamp?"="Time Stamp?") -> ("error out"=w2471:errorcluster)  [unwired: 7 in, 1 out]
        n1384 = local read "Phasor Grids"() -> (w2461:i32)
        n1385 = local read "ROI Cluster"() -> (w2453:T9)
        n1386 = local read "G_max"() -> (w2459:dbl)
        n1387 = local read "G_min"() -> (w2458:dbl)
        n1388 = local read "S_max"() -> (w2457:dbl)
        n1389 = local read "S_min"() -> (w2456:dbl)
        n1390 = flat-sequence {
          tunnel: w2454 -> [w2520]
          tunnel: [w2520] -> w2484
          frame #0 {
            n1391 = local write "Save 2D Images"(FALSE ("Save 3D Stacks")) -> ()
          }
        }
        n1392 = call "SaveMatrix.vi"("Experiment Name"="Experiment Name (2D)", "Identify Name"="Mix4" ("string"), "Data"=w2467, "error in"=w2471, "File Name"="File Name (2D)", "Index Name"=w2436, "path"=w2450, "Specify Range?"=FALSE ("Bound Pixel Value?"), "Enable?"="4 Mix?", "Crop Pixels"="Crop Pixels", "Time Stamp?"="Time Stamp?") -> ("error out"=w2465:errorcluster)  [unwired: 7 in, 1 out]
        n1393 = call "SavePhasor.vi"("Intensity"=w2441, "G Data"=w2448, "S Data"=w2447, "Threshold (max)"=w2439, "Threshold (min)"=w2438, "Auto Scale?"=FALSE, "Phasor Grids"=w2461, "error in"=w2465, "G_max"=w2459, "Index Name"=w2436, "G_min"=w2458, "S_max"=w2457, "Enable?"="Phasor?", "S_min"=w2456, "Time Stamp?"="Time Stamp?", "path"=w2450, "Experiment Name"="Experiment Name (2D)", "File Name"="File Name (2D)", "Identify Name"="Phasor" ("string"), "Crop Pixels"="Crop Pixels") -> ("error out"=w2455:errorcluster)  [unwired: 6 in, 1 out]
        n1394 = call "SaveOverlap.vi"("ROI Cluster"=w2453, "Intensity"=w2441, "Auto Scale?"=FALSE, "Threshold (max)"=w2439, "Threshold (min)"=w2438, "G Data"=w2448, "S Data"=w2447, "error in"=w2455, "File Name"="File Name (2D)", "Index Name"=w2436, "Experiment Name"="Experiment Name (2D)", "Time Stamp?"="Time Stamp?", "Identify Name"="Overlap" ("string"), "Enable?"="Overlap?", "path"=w2450, "Crop Pixels"="Crop Pixels") -> ("error out"=w2454:errorcluster)  [unwired: 10 in, 1 out]
      }
      event "Current Directory (2D)?": Value Change {
        n1395 = event-data() -> ()  [unwired: 1 in, 1 out]
        n1396 = case shown="True" "Current Directory (2D)?" {
          frame False {
          }
          frame True {
            n1397 = Current VI's Path() -> (path=w2530:path)
            n1398 = Strip Path(path=w2530) -> (stripped path=w2529:path)  [unwired: 1 out]
            n1399 = local write "Save Directory (2D)"(w2529) -> ()
          }
        }
      }
      event "Shutter": Value Change {
        n1400 = event-data() -> ()  [unwired: 1 in, 1 out]
        n1401 = local read "Shutter Line"() -> (w2531:tag)
        n1402 = call "ShutterControl.vi"("error in"=w2536, "Shutter Line"=w2531, "Shutter"="Shutter") -> ("error out"=w2535:errorcluster)  [unwired: 7 in, 1 out]
      }
      event "Power Rotate": Value Change {
        n1403 = event-data() -> ()  [unwired: 1 in, 1 out]
        n1404 = call "PowerControl.vi"("PowerControlPulseCounter"="Power Control Counter", "PowerControlDirectionLine"="Power Control Direction", "error in"=w2545, "Pulses\n(/0.45°)"="Pulses\n(/0.45deg)", "Direction"="Direction") -> ("error out"=w2544:errorcluster)  [unwired: 6 in]
      }
      event "Stop": Value Change {
        n1405 = event-data() -> ()  [unwired: 1 in, 1 out]
        n1406 = local read "Shutter Line"() -> (w2547:tag)
        n1407 = call "ShutterControl.vi"("error in"=w2556, "Shutter Line"=w2547, "Shutter"=FALSE) -> ("error out"=w2555:errorcluster, "Status Indicator"=w2551:bool)  [unwired: 7 in]
        n1408 = local write "Shutter"(w2551) -> ()
        n1409 = local write "Fast Scan Progress"(0.0 ("Fast Scan Progress")) -> ()
        n1410 = local write "Meas Progress"(0.0 ("Fast Scan Progress")) -> ()
        n1411 = local write "Measure"(FALSE ("Fast Scan")) -> ()
        n1412 = local write "Fast Scan"(FALSE ("Fast Scan")) -> ()
      }
      event "X+": Value Change {
        n1413 = event-data() -> ()  [unwired: 1 in, 1 out]
        n1414 = local read "Use Stage?"() -> (w2561:bool)
        n1415 = case shown="True" w2561 {
          tunnel: w2565 -> [w2567 w2583]
          tunnel: w2564 -> [w2566 w2582]
          tunnel: [w2566 w2569] -> w2559
          tunnel: [w2567 w2570] -> w2560
          frame False {
          }
          frame True {
            w2576 = "," ("string")
            n1416 = Number To Decimal String(number="XY Step (um)") -> (decimal integer string=w2575:string)  [unwired: 1 in]
            n1417 = Concatenate Strings("X" ("string"), w2576, w2575, w2576, w2575, "\r", "R" ("string")) -> (w2574:string)
            n1418 = VISA Write(VISA resource name=w2583, write buffer=w2574, error in (no error)=w2582) -> (VISA resource name out=w2581:refnum<visa-resource-name>, error out=w2580:errorcluster)  [unwired: 1 out]
            n1419 = VISA Read(VISA resource name=w2581, byte count=u32 256, error in (no error)=w2580) -> (VISA resource name out=w2571:refnum<visa-resource-name>, error out=w2568:errorcluster)  [unwired: 2 out]
            n1420 = VISA Clear(VISA resource name=w2571, error in (no error)=w2568) -> (VISA resource name out=w2570:refnum<visa-resource-name>, error out=w2569:errorcluster)
          }
        }
      }
      event "X-": Value Change {
        n1421 = event-data() -> ()  [unwired: 1 in, 1 out]
        n1422 = local read "Use Stage?"() -> (w2586:bool)
        n1423 = case shown="True" w2586 {
          tunnel: w2590 -> [w2592 w2608]
          tunnel: w2589 -> [w2591 w2607]
          tunnel: [w2592 w2595] -> w2585
          tunnel: [w2591 w2594] -> w2584
          frame False {
          }
          frame True {
            w2601 = "," ("string")
            n1424 = local read "XY Step (um)"() -> (w2603:u32)
            n1425 = Number To Decimal String(number=w2603) -> (decimal integer string=w2600:string)  [unwired: 1 in]
            n1426 = Concatenate Strings("X" ("string"), w2601, w2600, w2601, w2600, "\r", "L" ("string")) -> (w2597:string)
            n1427 = VISA Write(VISA resource name=w2608, write buffer=w2597, error in (no error)=w2607) -> (VISA resource name out=w2606:refnum<visa-resource-name>, error out=w2605:errorcluster)  [unwired: 1 out]
            n1428 = VISA Read(VISA resource name=w2606, byte count=u32 256, error in (no error)=w2605) -> (VISA resource name out=w2596:refnum<visa-resource-name>, error out=w2593:errorcluster)  [unwired: 2 out]
            n1429 = VISA Clear(VISA resource name=w2596, error in (no error)=w2593) -> (VISA resource name out=w2595:refnum<visa-resource-name>, error out=w2594:errorcluster)
          }
        }
      }
      event "Y+": Value Change {
        n1430 = event-data() -> ()  [unwired: 1 in, 1 out]
        n1431 = local read "Use Stage?"() -> (w2611:bool)
        n1432 = case shown="True" w2611 {
          tunnel: w2615 -> [w2617 w2633]
          tunnel: w2614 -> [w2616 w2632]
          tunnel: [w2616 w2619] -> w2609
          tunnel: [w2617 w2620] -> w2610
          frame False {
          }
          frame True {
            w2626 = "," ("string")
            n1433 = local read "XY Step (um)"() -> (w2628:u32)
            n1434 = Number To Decimal String(number=w2628) -> (decimal integer string=w2625:string)  [unwired: 1 in]
            n1435 = Concatenate Strings("X" ("string"), w2626, w2625, w2626, w2625, "\r", "F" ("string")) -> (w2622:string)
            n1436 = VISA Write(VISA resource name=w2633, write buffer=w2622, error in (no error)=w2632) -> (VISA resource name out=w2630:refnum<visa-resource-name>, error out=w2629:errorcluster)  [unwired: 1 out]
            n1437 = VISA Read(VISA resource name=w2630, byte count=u32 256, error in (no error)=w2629) -> (VISA resource name out=w2621:refnum<visa-resource-name>, error out=w2618:errorcluster)  [unwired: 2 out]
            n1438 = VISA Clear(VISA resource name=w2621, error in (no error)=w2618) -> (VISA resource name out=w2620:refnum<visa-resource-name>, error out=w2619:errorcluster)
          }
        }
      }
      event "Y-": Value Change {
        n1439 = event-data() -> ()  [unwired: 1 in, 1 out]
        n1440 = local read "Use Stage?"() -> (w2636:bool)
        n1441 = case shown="True" w2636 {
          tunnel: w2640 -> [w2642 w2658]
          tunnel: w2639 -> [w2641 w2657]
          tunnel: [w2642 w2645] -> w2635
          tunnel: [w2641 w2644] -> w2634
          frame False {
          }
          frame True {
            w2651 = "," ("string")
            n1442 = local read "XY Step (um)"() -> (w2653:u32)
            n1443 = Number To Decimal String(number=w2653) -> (decimal integer string=w2650:string)  [unwired: 1 in]
            n1444 = Concatenate Strings("X" ("string"), w2651, w2650, w2651, w2650, "\r", "B" ("string")) -> (w2647:string)
            n1445 = VISA Write(VISA resource name=w2658, write buffer=w2647, error in (no error)=w2657) -> (VISA resource name out=w2655:refnum<visa-resource-name>, error out=w2654:errorcluster)  [unwired: 1 out]
            n1446 = VISA Read(VISA resource name=w2655, byte count=u32 256, error in (no error)=w2654) -> (VISA resource name out=w2646:refnum<visa-resource-name>, error out=w2643:errorcluster)  [unwired: 2 out]
            n1447 = VISA Clear(VISA resource name=w2646, error in (no error)=w2643) -> (VISA resource name out=w2645:refnum<visa-resource-name>, error out=w2644:errorcluster)
          }
        }
      }
      event "Z+": Value Change {
        n1448 = event-data() -> ()  [unwired: 1 in, 1 out]
        n1449 = local read "Use Stage?"() -> (w2661:bool)
        n1450 = case shown="True" w2661 {
          tunnel: [w2666 w2669] -> w2659
          tunnel: [w2667 w2670] -> w2660
          tunnel: w2663 -> [w2667 w2673]
          tunnel: w2662 -> [w2666 w2672]
          frame False {
          }
          frame True {
            n1451 = Number To Decimal String(number="Z Step (.1um)") -> (decimal integer string=w2678:string)  [unwired: 1 in]
            n1452 = Concatenate Strings("C" ("string"), "," ("string"), w2678, "\r", "U" ("string")) -> (w2674:string)
            n1453 = VISA Write(VISA resource name=w2673, write buffer=w2674, error in (no error)=w2672) -> (VISA resource name out=w2682:refnum<visa-resource-name>, error out=w2681:errorcluster)  [unwired: 1 out]
            n1454 = VISA Read(VISA resource name=w2682, byte count=u32 256, error in (no error)=w2681) -> (VISA resource name out=w2671:refnum<visa-resource-name>, error out=w2668:errorcluster)  [unwired: 2 out]
            n1455 = VISA Clear(VISA resource name=w2671, error in (no error)=w2668) -> (VISA resource name out=w2670:refnum<visa-resource-name>, error out=w2669:errorcluster)
          }
        }
      }
      event "Z-": Value Change {
        n1456 = event-data() -> ()  [unwired: 1 in, 1 out]
        n1457 = local read "Use Stage?"() -> (w2686:bool)
        n1458 = case shown="True" w2686 {
          tunnel: [w2691 w2694] -> w2684
          tunnel: [w2692 w2695] -> w2685
          tunnel: w2688 -> [w2692 w2698]
          tunnel: w2687 -> [w2691 w2697]
          frame False {
          }
          frame True {
            n1459 = local read "Z Step (.1um)"() -> (w2699:u32)
            n1460 = Number To Decimal String(number=w2699) -> (decimal integer string=w2703:string)  [unwired: 1 in]
            n1461 = Concatenate Strings("C" ("string"), "," ("string"), w2703, "\r", "D" ("string")) -> (w2700:string)
            n1462 = VISA Write(VISA resource name=w2698, write buffer=w2700, error in (no error)=w2697) -> (VISA resource name out=w2707:refnum<visa-resource-name>, error out=w2706:errorcluster)  [unwired: 1 out]
            n1463 = VISA Read(VISA resource name=w2707, byte count=u32 256, error in (no error)=w2706) -> (VISA resource name out=w2696:refnum<visa-resource-name>, error out=w2693:errorcluster)  [unwired: 2 out]
            n1464 = VISA Clear(VISA resource name=w2696, error in (no error)=w2693) -> (VISA resource name out=w2695:refnum<visa-resource-name>, error out=w2694:errorcluster)
          }
        }
      }
      event "XY0": Value Change {
        n1465 = event-data() -> ()  [unwired: 1 in, 1 out]
        n1466 = local read "Use Stage?"() -> (w2711:bool)
        n1467 = case shown="True" w2711 {
          tunnel: w2715 -> [w2717 w2727]
          tunnel: w2714 -> [w2716 w2726]
          tunnel: [w2716 w2718] -> w2709
          tunnel: [w2717 w2720] -> w2710
          frame False {
          }
          frame True {
            n1468 = VISA Write(VISA resource name=w2727, write buffer="G,0,0" ("string"), error in (no error)=w2726) -> (VISA resource name out=w2723:refnum<visa-resource-name>, error out=w2722:errorcluster)  [unwired: 1 out]
            n1469 = VISA Read(VISA resource name=w2723, byte count=u32 256, error in (no error)=w2722) -> (VISA resource name out=w2721:refnum<visa-resource-name>, error out=w2719:errorcluster)  [unwired: 2 out]
            n1470 = VISA Clear(VISA resource name=w2721, error in (no error)=w2719) -> (VISA resource name out=w2720:refnum<visa-resource-name>, error out=w2718:errorcluster)
          }
        }
      }
      event "Z0": Value Change {
        n1471 = event-data() -> ()  [unwired: 1 in, 1 out]
        n1472 = local read "Use Stage?"() -> (w2730:bool)
        n1473 = case shown="True" w2730 {
          tunnel: w2734 -> [w2736 w2744]
          tunnel: w2733 -> [w2735 w2743]
          tunnel: [w2736 w2739] -> w2729
          tunnel: [w2735 w2738] -> w2728
          frame False {
          }
          frame True {
            n1474 = VISA Write(VISA resource name=w2744, write buffer="V,0" ("string"), error in (no error)=w2743) -> (VISA resource name out=w2742:refnum<visa-resource-name>, error out=w2741:errorcluster)  [unwired: 1 out]
            n1475 = VISA Read(VISA resource name=w2742, byte count=u32 256, error in (no error)=w2741) -> (VISA resource name out=w2740:refnum<visa-resource-name>, error out=w2737:errorcluster)  [unwired: 2 out]
            n1476 = VISA Clear(VISA resource name=w2740, error in (no error)=w2737) -> (VISA resource name out=w2739:refnum<visa-resource-name>, error out=w2738:errorcluster)
          }
        }
      }
      event "Go to Any XYZ": Value Change {
        n1477 = event-data() -> ()  [unwired: 1 in, 1 out]
        n1478 = local read "Use Stage?"() -> (w2749:bool)
        n1479 = case shown="True" w2749 {
          tunnel: w2753 -> [w2755 w2772]
          tunnel: w2752 -> [w2754 w2771]
          tunnel: [w2754 w2756] -> w2747
          tunnel: [w2755 w2757] -> w2748
          frame False {
          }
          frame True {
            w2767 = "," ("string")
            n1480 = Number To Decimal String(number="X Goal (um)") -> (decimal integer string=w2769:string)  [unwired: 1 in]
            n1481 = Number To Decimal String(number="Y Goal (um)") -> (decimal integer string=w2766:string)  [unwired: 1 in]
            n1482 = Number To Decimal String(number="Z Goal (.1um)") -> (decimal integer string=w2765:string)  [unwired: 1 in]
            n1483 = Concatenate Strings("G" ("string"), w2767, w2769, w2767, w2766, w2767, w2765) -> (w2768:string)
            n1484 = VISA Write(VISA resource name=w2772, write buffer=w2768, error in (no error)=w2771) -> (VISA resource name out=w2761:refnum<visa-resource-name>, error out=w2760:errorcluster)  [unwired: 1 out]
            n1485 = VISA Read(VISA resource name=w2761, byte count=u32 256, error in (no error)=w2760) -> (VISA resource name out=w2759:refnum<visa-resource-name>, error out=w2758:errorcluster)  [unwired: 2 out]
            n1486 = VISA Clear(VISA resource name=w2759, error in (no error)=w2758) -> (VISA resource name out=w2757:refnum<visa-resource-name>, error out=w2756:errorcluster)